vi "Configured Acquisition Trigger (Host)_20221111.vi"() -> ()   [LabVIEW 2021]
doc: "Use this VI as a template to design an application that acquires data using advanced triggering logic from the NI PXIe-5170R/5171R."
uses:
  <instrlib>/_niInstr/Multirecord Acquisition/Interface/v1/Host/Public/Requested Record Info.ctl
  <instrlib>/HSAI-RIO/Types/v1/Host/Typedefs/Temp Source.ctl
  <vilib>/FPGAPlugInAG/PXIe-5172 (8CH - 410T)/niLvFpga_Open_PXIe-5172 (8CH - 410T).vi
  <vilib>/rvi/interface/common/dynamic/niFpgaDynamicAddResources.vi
  <vilib>/FPGAPlugInAG/Dynamic/niLvFpga_Close_Dynamic.vi
  <vilib>/rvi/interface/nirviOpenFPGA/nirviOpenFPGA.xnode
  FPGA Bitfiles/Multirecord Acquisition FPGA_20221228a.lvbitx
  <vilib>/rvi/interface/nirviCloseFPGA/nirviCloseFPGA.xnode
  Device Session/Device Session.lvclass
  <instrlib>/HSAI-RIO/Types/v1/Host/niHSAI Types v1 Host.lvlib
  <instrlib>/_niInstr/Multirecord Acquisition/Interface/v1/Host/niInstr Multirecord Acquisition v1 Host.lvclass
panel:
  out "requested record info":T1={"number of samples"=0, "starting sample number"=0, "number of channels"=1, "timestamps"=[]}
  out "TrigCfg 0":T2
  in  "ResetTrig":bool=TRUE
  in  "Sliding Window Trigger":cluster{"Range":dbl, "StartCenter":dbl}[](array[cluster])=[{"Range"=2.01, "StartCenter"=0.0}, {"Range"=0.01, "StartCenter"=1.0}, {"Range"=5.0, "StartCenter"=0.0}, {"Range"=5.0, "StartCenter"=0.0}, {"Range"=5.0, "StartCenter"=0.0}, {"Range"=5.0, "StartCenter"=0.0}, {"Range"=5.0, "StartCenter"=0.0}, {"Range"=5.0, "StartCenter"=0.0}]
  out "actual sample rate":dbl format="%#_6p"
  in  "onboard sample clock rate":dbl(ring)=200000000.0 items=["250 MHz"=250000000.0, "200 MHz"=200000000.0, "150 MHz"=150000000.0]
  in  "impedance":enum8{"Default", "1 mega ohm", "50 ohm"}(ring)
  in  "vertical offset (V)":dbl format="%.2p"
  out "Waveform Graph":T3(graph)
  out "fpga temperature (°C)":dbl(slide)=60.0 scale=0.0..96.0 scale format="%#_6p"
  out "power consumption (W)":dbl(slide)=20.0 scale=0.0..38.25 scale format="%#_6p"
  in  "mode":T4(ring)=enum."OR"
  in  "decimation factor":u16=1
  in  "coupling":enum8{"Default", "DC", "AC"}(ring)
  in  "bandwidth":T5(ring)
  in  "pretrigger samples":u64=500
  in  "number of samples":u64=1000
  in  "RIO Device":tag="PXI2Slot3"
  in  "channel(s)":string="0"
  in  "timeout (ms)":i32=5000
  in  "vertical range (Vpp)":dbl=1.0 format="%.2p"
  out "error out":errorcluster
  in  "stop":bool
  # "RIO Device"
  # "Vertical Settings"
  # "Trigger Settings"
  # "System Monitor"
  # "Acquisition Settings"
  # "Clocking"
  # "DSP"
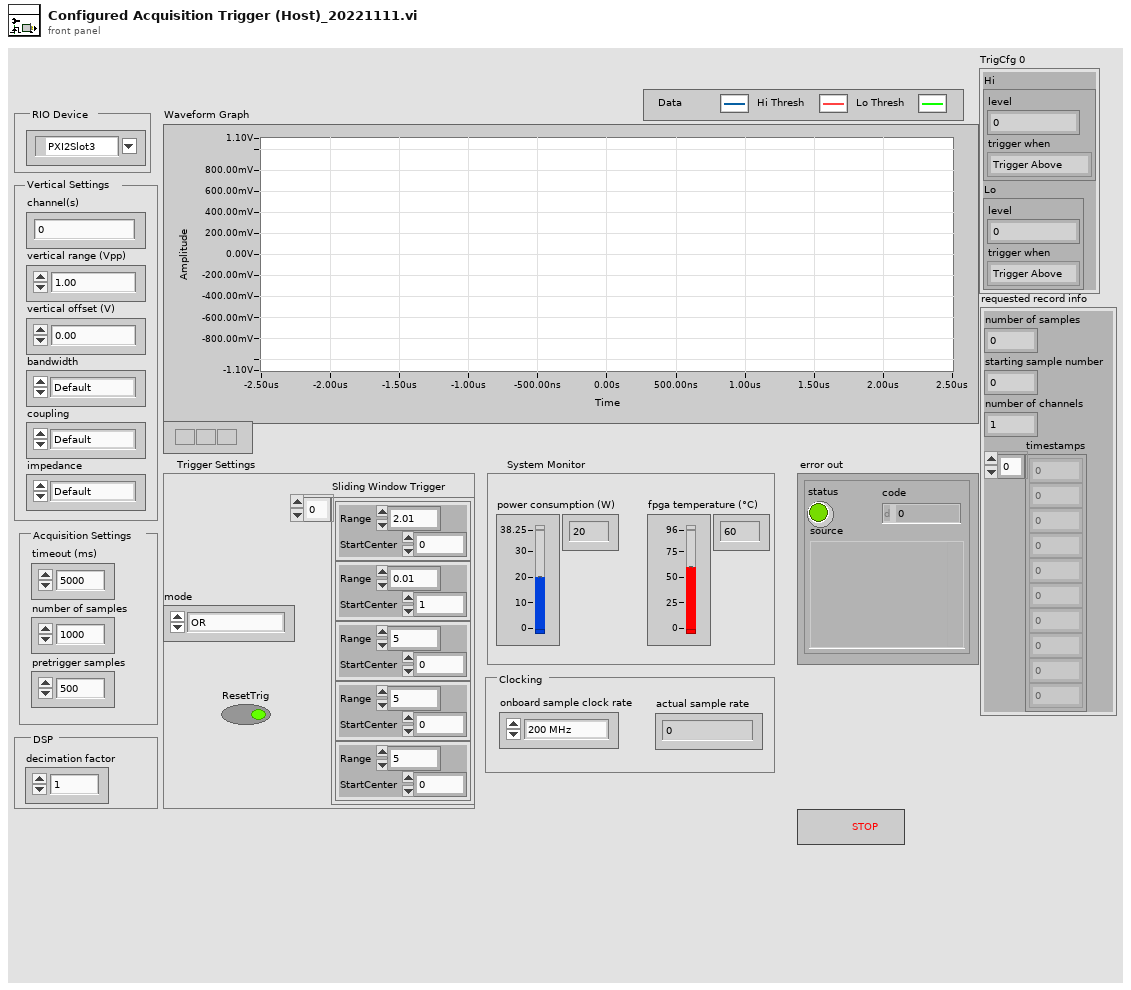
[diagram p1: front panel]
types:
  T1 = typedef "niInstr Multirecord Acquisition v1 Host.lvclass/Requested Record Info.ctl" = cluster{"number of samples":u64, "starting sample number":u64, "number of channels":u64, "timestamps":u64[]}
  T2 = cluster{"Hi":cluster{"level":fxp<+/-,18,1>, "trigger when":enum8{"Trigger Above", "Trigger Below"}}, "Lo":cluster{"level":fxp<+/-,18,1>, "trigger when":enum8{"Trigger Above", "Trigger Below"}}}
  T3 = cluster{"relativeX":dbl, "sample rate":dbl, "data in":dbl[]}[]
  T4 = enum16{"Immediate", "A", "B", "OR", "AND", "A THEN B", "B THEN A", "High Resolution"}
  T5 = enum8{"Default", "Full Bandwidth", "Anti-alias Filter", "80 MHz FIR Filter", "40 MHz FIR Filter", "20 MHz FIR Filter"}
  T6 = typedef "niHSAI Types v1 Host.lvlib/Temp Source.ctl" = enum8{"Device Temperature", "Thermal Shutdown Margin", "FPGA Temperature", "FPGA Temperature Limit"}
  T7 = typedef "niInstr Multirecord Acquisition v1 Host.lvclass/Scaling Coefficient.ctl" = cluster{"gain":dbl, "offset":dbl}
  T8 = typedef "ChannelWindowClust.ctl" = cluster{"HalfRange":fxp<+/-,18,5>, "StartCenter":fxp<+/-,18,5>}
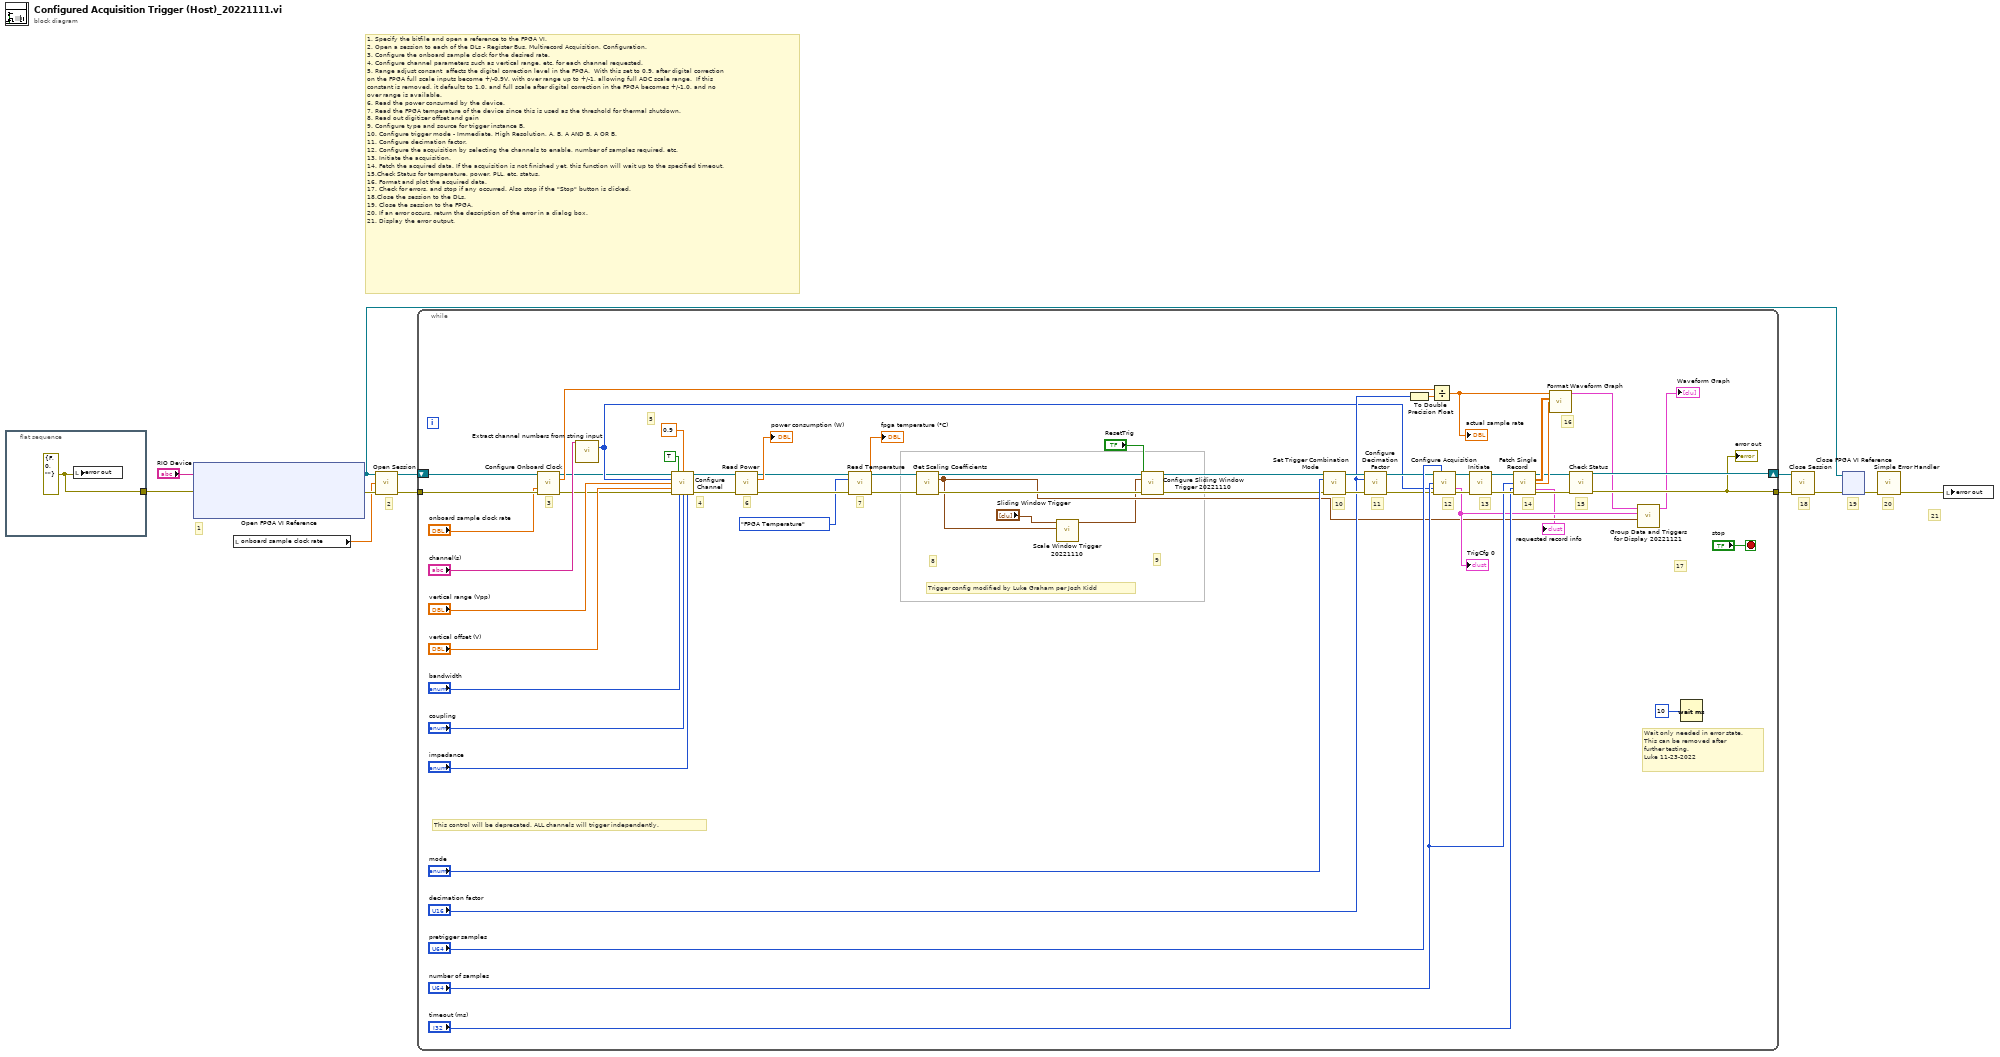
[diagram p0: block diagram]
diagram:
  # "21"
  # "20"
  # "19"
  # "18"
  # "1. Specify the bitfile and open a reference to the FPGA VI.\n2. Open a session to each of the DLs - Register Bus, Multirecord Acquisition, Configuration.\n3. Configure the onboard sample clock for the desired rate.\n4. Configure channel parameters such as vertical range, etc. for each channel requested.\n5. Range adjust consant  affects the digital correction level in the FPGA.  With this set to 0.9, after digital correction\non the FPGA full scale inputs become +/-0.9V, with over range up to +/-1, allowing full ADC scale range.  If this \nconstant is removed, it defaults to 1.0, and full scale after digital correction in the FPGA becomes +/-1.0, and no\nover range is available.  \n6. Read the power consumed by the device.\n7. Read the FPGA temperature of the device since this is used as the threshold for thermal shutdown.\n8. Read out digitizer offset and gain\n9. Configure type and source for trigger instance B.\n10. Configure trigger mode - Immediate, High Resolution, A, B, A AND B, A OR B.\n11. Configure decimation factor.\n12. Configure the acquisition by selecting the channels to enable, number of samples required, etc.\n13. Initiate the acquisition.\n14. Fetch the acquired data. If the acquisition is not finished yet, this function will wait up to the specified timeout.\n15.Check Status for temperature, power, PLL, etc. status. \n16. Format and plot the acquired data.\n17. Check for errors, and stop if any occurred. Also stop if the \"Stop\" button is clicked.\n18.Close the session to the DLs.\n19. Close the session to the FPGA.\n20. If an error occurs, return the description of the error in a dialog box.\n21. Display the error output."
  # "2"
  # "1"
  n1 = flat-sequence {
    tunnel: [w13] -> w1
    frame #0 {
      w13 = errorcluster {"status"=FALSE, "code"=0, "source"=""} ("error constant")
      n2 = local write "error out"(w13) -> ()
    }
  }
  n3 = xnode "Open FPGA VI Reference"("error in"=w1, "resource name"="RIO Device") -> ("FPGA VI Reference Out"=w5:refnum<k20>, "error out"=w7:errorcluster)
  n4 = local read "onboard sample clock rate"() -> (w3:dbl)
  n5 = call "Open Session.vi"("FPGA VI Ref"=w5, "adc clock rate (Hz)"=w3, "error in"=w7) -> ("device session out"=w10:refnum<class "Device Session.lvclass">, "error out"=w9:errorcluster)  [unwired: 11 in]
  n6 = while {
    shift-right: [w45] -> w11
    shift-left: w10 -> [w58]
    tunnel: w9 -> [w57]
    tunnel: [w20] -> w12
    stop <- "stop" stop-if-true
    # "Wait only needed in error state.\nThis can be removed after\nfurther testing.\nLuke 11-23-2022"
    # "This control will be deprecated. ALL channels will trigger independently."
    # "Trigger config modified by Luke Graham per Josh Kidd"
    # "4"
    # "5"
    # "7"
    # "6"
    # "15"
    # "11"
    # "3"
    # "17"
    # "16"
    # "10"
    # "9"
    # "8"
    # "14"
    # "13"
    # "12"
    n7 = call "Configure Onboard Clock.vi"("device session in"=w58, "adc clock rate (Hz)"="onboard sample clock rate", "error in"=w57) -> ("device session out"=w22:refnum<class "Device Session.lvclass">, "actual adc clock rate (Hz)"=w49:dbl, "error out"=w56:errorcluster)  [unwired: 9 in, 1 out]
    n8 = call "Extract channel numbers from string input.vi"("channel input"="channel(s)") -> ("array of chans"=w30:u32[])  [unwired: 13 in, 1 out]
    n9 = call "Configure Channel.vi"("device session in"=w22, "enable channel (T)"=TRUE ("enable channel"), "range adjust"=0.9, "channels"=w30, "vertical range (Vpp)"="vertical range (Vpp)", "vertical offset (V)"="vertical offset (V)", "error in"=w56, "bandwidth"="bandwidth", "coupling"="coupling", "impedance"="impedance") -> ("device session out"=w40:refnum<class "Device Session.lvclass">, "error out"=w39:errorcluster)  [unwired: 4 in]
    n10 = call "Read Power.vi"("device session in"=w40, "error in"=w39) -> ("device session out"=w41:refnum<class "Device Session.lvclass">, "power (W)"=→"power consumption (W)":dbl, "error out"=w42:errorcluster)  [unwired: 11 in]
    n11 = call "Read Temperature.vi"("device session in"=w41, "source"=Temp_Source."FPGA Temperature", "error in"=w42) -> ("device session out"=w29:refnum<class "Device Session.lvclass">, "temperature (°C)"=→"fpga temperature (°C)":dbl, "error out"=w28:errorcluster)  [unwired: 10 in]
    n12 = call "Get Scaling Coefficients.vi"("device session in"=w29, "error in"=w28) -> ("device session out"=w26:refnum<class "Device Session.lvclass">, "scaling coefficients"=w16:T7[], "error out"=w24:errorcluster)  [unwired: 11 in]
    n13 = call "Scale Window Trigger 20221110.vi"("scaling coefficients"=w16, "Sliding Window Trigger"="Sliding Window Trigger") -> ("Sliding Window Trigger (FXP)"=w15:T8[])  [unwired: 9 in]
    n14 = call "Configure Sliding Window Trigger 20221110.vi"("device session in"=w26, "Sliding Window Triggers (FXP)"=w15, "ResetTrig"="ResetTrig", "error in"=w24) -> ("device session out"=w25:refnum<class "Device Session.lvclass">, "error out"=w23:errorcluster)  [unwired: 10 in]
    n15 = call "Set Trigger Combination Mode.vi"("device session in"=w25, "mode"="mode", "error in"=w23) -> ("device session out"=w54:refnum<class "Device Session.lvclass">, "error out"=w53:errorcluster)  [unwired: 11 in]
    n16 = call "Configure Decimation Factor.vi"("device session in"=w54, "decimation factor"="decimation factor", "error in"=w53) -> ("device session out"=w51:refnum<class "Device Session.lvclass">, "error out"=w52:errorcluster)  [unwired: 11 in]
    n17 = To Double Precision Float(number="decimation factor") -> (double precision float=w55:dbl)
    n18 = Divide(x=w49, y=w55) -> (x/y=w32:dbl)
    "actual sample rate" <- w32
    n19 = call "Configure Acquisition.vi"("device session in"=w51, "pretrigger samples"="pretrigger samples", "number of samples"="number of samples", "channels to store"=w30, "error in"=w52) -> ("device session out"=w68:refnum<class "Device Session.lvclass">, "TrigCfg 0"=w17:T2, "error out"=w71:errorcluster)  [unwired: 7 in, 1 out]
    "TrigCfg 0" <- w17
    n20 = call "Initiate.vi"("device session in"=w68, "error in"=w71) -> ("device session out"=w69:refnum<class "Device Session.lvclass">, "error out"=w70:errorcluster)  [unwired: 12 in]
    n21 = call "Fetch Single Record.vi"("device session in"=w69, "number of samples"="number of samples", "timeout (ms)"="timeout (ms)", "error in"=w70) -> ("device session out"=w46:refnum<class "Device Session.lvclass">, "data"=w60:dbl[][], "relativeX (samples)"=w59:dbl, "requested record info"=→"requested record info":T1, "error out"=w47:errorcluster)  [unwired: 7 in]
    n22 = call "Format Waveform Graph.vi"("sample rate (Hz)"=w32, "data in"=w60, "relativeX (samples)"=w59) -> ("waveform out"=w19:T3)  [unwired: 12 in]
    n23 = call "Check Status.vi"("device session in"=w46, "error in"=w47) -> ("device session out"=w45:refnum<class "Device Session.lvclass">, "error out"=w20:errorcluster)  [unwired: 12 in]
    "error out" <- w20
    n24 = call "Group Data and Triggers for Display 20221121.vi"("scaling coefficients"=w16, "TrigCfg 0"=w17, "Data waveform"=w19) -> ("Data for Display"=→"Waveform Graph":T3)  [unwired: 8 in]
    n25 = Wait (ms)(milliseconds to wait=u32 10) -> ()  [unwired: 1 out]
  }
  n26 = call "Close Session.vi"("device session in"=w11, "error in"=w12) -> ("error out"=w6:errorcluster)  [unwired: 13 in]
  n27 = xnode "Close FPGA VI Reference"("FPGA VI Reference In"=w5, "error in"=w6) -> ("error out"=w4:errorcluster)
  n28 = call <vilib>:"Simple Error Handler.vi"("error in (no error)"=w4) -> ("error out"=w2:errorcluster)  [unwired: 4 in, 4 out]
  n29 = local write "error out"(w2) -> ()
